vi "HFRR ADV v041.vi"() -> ()   [LabVIEW 2025] (continued)
                    n294 = call "ELAPSED TIMER VI - abort test.vi"("TARGET"=60.0, "RESET"=w401, "PAUSE"=FALSE) -> ("ELAPSED INDICATION"=w399:bool)  [unwired: 6 in, 2 out]
                    n295 = case shown="True" w399 {
                      frame False {
                      }
                      frame True {
                        n296 = stacked-sequence {
                          frame #0 {
                            w404 = FALSE
                            n297 = local write "RUN"(w404) -> ()
                            n298 = local write "Auto Start Test"(w404) -> ()
                          }
                          frame #1 {
                            n299 = One Button Dialog(message="Test stopped due to a communication error. Reconnect the C1 and C2 cables.") -> ()  [unwired: 1 in, 1 out]
                          }
                        }
                      }
                    }
                  }
                }
              }
            }
          }
          frame Enabled {
          }
        }
        n300 = Get Date/Time In Seconds() -> (seconds since 1Jan1904=w385:timestamp)
        n301 = Format Into String(format string="%<%I:%M:%S:%p %d:%B:%Y>T", w385) -> (resulting string=→"Time Stamp":string)  [unwired: 2 in, 1 out]
        n302 = local read "Service Password enable"() -> (w377:bool)
        n303 = local read "FILE"() -> (w382:string)
        n304 = call <vilib>:"Trim Whitespace.vi"("string"=w382) -> ("trimmed string"=w381:string)  [unwired: 1 in]
        n305 = String Length(string=w381) -> (length=w380:i32)
        n306 = Greater?(x=w380, y=1) -> (0:w378:bool)
        n307 = case shown="False" w378 {
          tunnel: w377 -> [w406 _]
          frame False {
            n308 = case shown="False" w406 {
              frame True {
                w407 = "Test Start In Service Mode" ("Tip Strip")
                w408 = T19."Enabled" ("Disabled")
                n309 = property on="Auto Start Test" class="Bool (strict)"("DisabledEnum"=w408, "TipStrip"=w407) -> ()  [unwired: 2 in, 2 out]
                n310 = property on="RUN" class="Bool (strict)"("DisabledEnum"=w408, "TipStrip"=w407) -> ()  [unwired: 2 in, 2 out]
              }
              frame False {
                w409 = "Enter File Name to Start Test" ("Tip Strip")
                w410 = T19."Disabled and Grayed Out" ("Disabled")
                n311 = property on="Auto Start Test" class="Bool (strict)"("DisabledEnum"=w410, "TipStrip"=w409) -> ()  [unwired: 2 in, 2 out]
                n312 = property on="RUN" class="Bool (strict)"("DisabledEnum"=w410, "TipStrip"=w409) -> ()  [unwired: 2 in, 2 out]
              }
            }
          }
          frame True {
            w411 = "" ("Tip Strip")
            w412 = T19."Enabled" ("Disabled")
            n313 = property on="Auto Start Test" class="Bool (strict)"("DisabledEnum"=w412, "TipStrip"=w411) -> ()  [unwired: 2 in, 2 out]
            n314 = property on="RUN" class="Bool (strict)"("DisabledEnum"=w412, "TipStrip"=w411) -> ()  [unwired: 2 in, 2 out]
          }
        }
      }
      event "RUN": Value Change {
        n315 = event-data() -> ()  [unwired: 1 in, 6 out]
        n316 = local read "RUN"() -> (w414:bool)
        n317 = case shown="False" w414 {
          frame False {
            n318 = flat-sequence {
              frame #0 {
                n319 = local write "START TEMP"(FALSE ("START TEMP")) -> ()
              }
              frame #1 {
                n320 = Wait (ms)(milliseconds to wait=u32 1500) -> ()  [unwired: 1 out]
              }
              frame #2 {
                n321 = local write "Humidity 2"(TRUE ("Humidity")) -> ()
              }
              frame #3 {
                n322 = local write "Due Write"("VC;0") -> ()
              }
              frame #4 {
                n323 = Wait (ms)(milliseconds to wait=u32 1500) -> ()  [unwired: 1 out]
              }
              frame #5 {
                w424 = T19."Enabled" ("Disabled")
                (unwired) T26."Imaging" ("Main Dashboard Buttons")
                (unwired) T21."Adv Scar" ("Main Tab")
                w426 = "" ("FILE")
                n324 = local write "measured_stroke"(0.0 ("measured_stroke")) -> ()
                n325 = local write "Due Write"("VC;0") -> ()
                n326 = local write "FILE"(w426) -> ()
                n327 = local write "Batch Ref Num :"(w426) -> ()
                n328 = local write "Fuel Discription :"(w426) -> ()
                n329 = local write "Main Tab"(T2."Adv Scar" ("Main Tab")) -> ()
                n330 = local write "Remarks :"(w426) -> ()
                n331 = local write "Main Dashboard Buttons"(T1."Imaging" ("Main Dashboard Buttons")) -> ()
                n332 = local write "TEST FILE NAM,E SAVED"(FALSE ("TEST FILE NAM,E SAVED")) -> ()
                n333 = property on="Stroke ( mm )" class="WFChart (strict)"("History Data"=cluster{"y":dbl, dbl, "y":dbl}[] []) -> ()  [unwired: 2 in, 2 out]
                n334 = property on="Auto Start Test" class="Bool (strict)"("Visible"=TRUE) -> ()  [unwired: 2 in, 2 out]
                n335 = property on="FRICVALZ 2" class="Bool (strict)"("DisabledEnum"=w424) -> ()  [unwired: 2 in, 2 out]
                n336 = property on="FRICVALZ 4" class="Bool (strict)"("DisabledEnum"=w424) -> ()  [unwired: 2 in, 2 out]
                n337 = property on="FRICVALZ 3" class="Bool (strict)"("DisabledEnum"=w424) -> ()  [unwired: 2 in, 2 out]
              }
            }
          }
          frame True {
            n338 = stacked-sequence {
              frame #0 {
                n339 = local write "Due Write"("DAC;200") -> ()
              }
              frame #1 {
                n340 = Wait (ms)(milliseconds to wait=u32 1500) -> ()  [unwired: 1 out]
              }
              frame #2 {
                n341 = local write "Due Write"("DAC;200") -> ()
              }
              frame #3 {
                n342 = Wait (ms)(milliseconds to wait=u32 1500) -> ()  [unwired: 1 out]
              }
              frame #4 {
                n343 = local write "Due Write"("VC;1") -> ()
              }
              frame #5 {
                n344 = Wait (ms)(milliseconds to wait=u32 2000) -> ()  [unwired: 1 out]
              }
              frame #6 {
                n345 = local write "Due Write"("VC;1") -> ()
              }
              frame #7 {
                n346 = Wait (ms)(milliseconds to wait=u32 2000) -> ()  [unwired: 1 out]
              }
              frame #8 {
                w438 = T19."Disabled" ("Disabled")
                n347 = property on="Auto Start Test" class="Bool (strict)"("Visible"=FALSE) -> ()  [unwired: 2 in, 2 out]
                n348 = local write "START TEMP"(TRUE ("START TEMP")) -> ()
                n349 = property on="FRICVALZ 2" class="Bool (strict)"("DisabledEnum"=w438) -> ()  [unwired: 2 in, 2 out]
                n350 = property on="FRICVALZ 4" class="Bool (strict)"("DisabledEnum"=w438) -> ()  [unwired: 2 in, 2 out]
                n351 = property on="FRICVALZ 3" class="Bool (strict)"("DisabledEnum"=w438) -> ()  [unwired: 2 in, 2 out]
              }
            }
          }
        }
      }
      event "run test Calibration": Value Change {
        n352 = event-data() -> ()  [unwired: 1 in, 6 out]
        n353 = local read "run test Calibration"() -> (w440:bool)
        n354 = case shown="True" w440 {
          frame False {
            n355 = flat-sequence {
              frame #0 {
                n356 = local write "START TEMP"(FALSE ("START TEMP")) -> ()
              }
              frame #1 {
                n357 = Wait (ms)(milliseconds to wait=u32 1500) -> ()  [unwired: 1 out]
              }
              frame #2 {
              }
              frame #3 {
                n358 = local write "Due Write"("VC;0") -> ()
              }
              frame #4 {
                n359 = Wait (ms)(milliseconds to wait=u32 1500) -> ()  [unwired: 1 out]
              }
              frame #5 {
                n360 = local write "Due Write"("VC;0") -> ()
                n361 = local write "Friction Force Calibration Result Tab"(enum32{"Calibration Results", "Page 2"}."Calibration Results" ("Friction Force Calibration Result Tab")) -> ()
                n362 = property on="Friction Force Calibration Result Tab" class="TabCtl (strict)"("Visible"=TRUE) -> ()  [unwired: 2 in, 2 out]
              }
            }
          }
          frame True {
            n363 = flat-sequence {
              frame #0 {
                n364 = local write "Due Write"("VC;1") -> ()
              }
              frame #1 {
                n365 = Wait (ms)(milliseconds to wait=u32 2000) -> ()  [unwired: 1 out]
              }
              frame #2 {
                n366 = local write "Due Write"("VC;1") -> ()
              }
              frame #3 {
                n367 = Wait (ms)(milliseconds to wait=u32 2000) -> ()  [unwired: 1 out]
              }
              frame #4 {
                n368 = local write "START TEMP"(TRUE ("START TEMP")) -> ()
                n369 = local write "Friction Force Calibration Result Tab"(enum32{"Calibration Results", "Page 2"}."Calibration Results" ("Friction Force Calibration Result Tab")) -> ()
                n370 = property on="Friction Force Calibration Result Tab" class="TabCtl (strict)"("Visible"=TRUE) -> ()  [unwired: 2 in, 2 out]
              }
            }
          }
        }
      }
      event "Auto": Value Change {
        n371 = event-data() -> ()  [unwired: 1 in, 6 out]
        n372 = stacked-sequence {
          frame #0 {
            n373 = local write "FILE"("") -> ()
          }
          frame #1 {
            n374 = Get Date/Time In Seconds() -> (seconds since 1Jan1904=w460:timestamp)
            n375 = Format Into String(format string="%<%I_%M_%S_%p_%d_%B_%Y>T", w460) -> (resulting string=w459:string)  [unwired: 2 in, 1 out]
            n376 = local write "FILE"(w459) -> ()
          }
        }
        n377 = local read "Auto"() -> (w457:bool)
        n378 = Not(x=w457) -> (.not. x?=w456:bool)
        n379 = local write "Auto"(w456) -> ()
      }
      event "Auto Start Temp": Value Change {
        n380 = event-data() -> ()  [unwired: 1 in, 6 out]
        n381 = local read "Auto Start Test"() -> (w463:bool)
        n382 = case shown="False" w463 {
          frame False {
            n383 = stacked-sequence {
              frame #0 {
                n384 = local write "START TEMP"(FALSE ("START TEMP")) -> ()
              }
              frame #1 {
                n385 = Wait (ms)(milliseconds to wait=u32 2000) -> ()  [unwired: 1 out]
              }
              frame #2 {
                n386 = local write "Due Write"("VC;0") -> ()
              }
              frame #3 {
                n387 = Wait (ms)(milliseconds to wait=u32 2000) -> ()  [unwired: 1 out]
              }
              frame #4 {
                w474 = T19."Enabled" ("Disabled")
                (unwired) T26."Imaging" ("Main Dashboard Buttons")
                w475 = "" ("FILE")
                n388 = local write "Main Tab"(T2."Adv Scar" ("Main Tab")) -> ()
                n389 = local write "measured_stroke"(0.0 ("measured_stroke")) -> ()
                n390 = local write "Main Dashboard Buttons"(T1."Imaging" ("Main Dashboard Buttons")) -> ()
                n391 = property on="RUN" class="Bool (strict)"("Visible"=TRUE) -> ()  [unwired: 2 in, 2 out]
                n392 = local write "Due Write"("VC;0") -> ()
                n393 = local write "Humidity 2"(TRUE ("Humidity")) -> ()
                n394 = local write "TEST FILE NAM,E SAVED"(FALSE ("TEST FILE NAM,E SAVED")) -> ()
                n395 = local write "Fuel Discription :"(w475) -> ()
                n396 = local write "Batch Ref Num :"(w475) -> ()
                n397 = local write "Remarks :"(w475) -> ()
                n398 = local write "FILE"(w475) -> ()
                n399 = property on="FRICVALZ 2" class="Bool (strict)"("DisabledEnum"=w474) -> ()  [unwired: 2 in, 2 out]
                n400 = property on="FRICVALZ 4" class="Bool (strict)"("DisabledEnum"=w474) -> ()  [unwired: 2 in, 2 out]
                n401 = property on="FRICVALZ 3" class="Bool (strict)"("DisabledEnum"=w474) -> ()  [unwired: 2 in, 2 out]
              }
            }
          }
          frame True {
            n402 = stacked-sequence {
              frame #0 {
                n403 = local write "Due Write"("DAC;200") -> ()
              }
              frame #1 {
                n404 = Wait (ms)(milliseconds to wait=u32 1500) -> ()  [unwired: 1 out]
              }
              frame #2 {
                n405 = local write "Due Write"("DAC;200") -> ()
              }
              frame #3 {
                n406 = Wait (ms)(milliseconds to wait=u32 1000) -> ()  [unwired: 1 out]
              }
              frame #4 {
                n407 = local write "Due Write"("VC;1") -> ()
              }
              frame #5 {
                n408 = Wait (ms)(milliseconds to wait=u32 2000) -> ()  [unwired: 1 out]
              }
              frame #6 {
                n409 = local write "Due Write"("VC;1") -> ()
              }
              frame #7 {
                n410 = Wait (ms)(milliseconds to wait=u32 2000) -> ()  [unwired: 1 out]
              }
              frame #8 {
                w486 = T19."Disabled" ("Disabled")
                n411 = property on="RUN" class="Bool (strict)"("Visible"=FALSE) -> ()  [unwired: 2 in, 2 out]
                n412 = property on="FRICVALZ 2" class="Bool (strict)"("DisabledEnum"=w486) -> ()  [unwired: 2 in, 2 out]
                n413 = property on="FRICVALZ 4" class="Bool (strict)"("DisabledEnum"=w486) -> ()  [unwired: 2 in, 2 out]
                n414 = property on="FRICVALZ 3" class="Bool (strict)"("DisabledEnum"=w486) -> ()  [unwired: 2 in, 2 out]
                "START TEMP" <- TRUE
              }
            }
          }
        }
      }
      event "FILE", "USERNAME", "USER ID": Mouse Enter {
        n415 = event-data() -> ()  [unwired: 1 in, 4 out]
        n416 = dll-call lib="kernel32.dll" fn="Wow64DisableWow64FsRedirection"("OldValue"=0) -> (error out=w493:errorcluster, "OldValue"=w491:i32)  [unwired: 4 in, 1 out]
        n417 = call <vilib>:"System Exec.vi"("run minimized? (F)"=TRUE, "error in (no error)"=w493, "command line"="C:\\Program Files\\Common Files\\Microsoft Shared\\Ink\\TabTip.exe") -> ("error out"=w492:errorcluster)  [unwired: 5 in, 3 out]
        n418 = dll-call lib="kernel32.dll" fn="Wow64EnableWow64FsRedirection"(error in=w492, "OldValue"=w491) -> ()  [unwired: 4 in, 2 out]
      }
      event "EDIT": Value Change {
        n419 = event-data() -> ()  [unwired: 1 in, 6 out]
        n420 = local read "EDIT"() -> (w494:bool)
        n421 = case shown="False" w494 {
          frame False {
            n422 = control-ref of="This VI"() -> (w511:refnum<vi>)
            n423 = property class="VI"(reference=w511) -> (reference out=w502:refnum<vi>, error out=w506:errorcluster, "Panel"=w510:refnum<vi>)  [unwired: 1 in]
            n424 = property class="Pnl"(reference=w510, error in=w506) -> (reference out=w504:refnum<vi>, error out=w507:errorcluster, "Panes[]"=w509:refnum<vi>[])
            n425 = for {
              tunnel: w509 -> [w517] mode=indexing
              tunnel: T24."Always Off" ("Horizontal Scrollbar Visibility") -> [w516]
              tunnel: w507 -> [w513]
              tunnel: [w512] -> w505
              n426 = property class="Pane"(reference=w517, error in=w513, "HorizScrollbarVisibility"=w516) -> (reference out=w514:refnum<vi>, error out=w515:errorcluster)
              n427 = Close Reference(reference=w514, error in (no error)=w515) -> (error out=w512:errorcluster)
            }
            n428 = Close Reference(reference=w504, error in (no error)=w505) -> (error out=w503:errorcluster)
            n429 = Close Reference(reference=w502, error in (no error)=w503) -> (error out=w497:errorcluster)
            "error out 7" <- w497
            n430 = call <vilib>:"Clear Errors.vi"("error in (no error)"=w497) -> ("error out"=w496:errorcluster)  [unwired: 5 in, 1 out]
            n431 = local write "Service Password enable"(FALSE ("Service Password enable")) -> ()
            n432 = call <userlib>:"Fit VI window to Largest Dec.vi"("error in (no error)"=w496, "border spacing (2 px)"=1) -> ("error out"=w501:errorcluster, "dup VI Ref"=w499:refnum<vi>)  [unwired: 4 in]
            n433 = invoke on="Invoke Node" class="VI" method="FP.Run-Time Position.Maximized"(reference=w499, error in=w501) -> (error out=w500:errorcluster)  [unwired: 2 in, 3 out]
            n434 = call <vilib>:"Clear Errors.vi"("error in (no error)"=w500) -> ()  [unwired: 5 in, 2 out]
          }
          frame True {
          }
        }
      }
      event "Heater Button": Value Change {
        n435 = event-data() -> ()  [unwired: 1 in, 6 out]
        n436 = local read "Heater Button"() -> (w518:bool)
        n437 = case shown="True" w518 {
          frame True {
            n438 = stacked-sequence {
              frame #0 {
                n439 = Wait (ms)(milliseconds to wait=u32 1500) -> ()  [unwired: 1 out]
              }
              frame #1 {
                n440 = local read "Set Temp"() -> (w520:dbl)
                n441 = Number To Fractional String(number=w520, precision (6)=i16 2) -> (F-format string=w523:string)  [unwired: 2 in]
                n442 = Concatenate Strings("ST;" ("Command"), w523) -> (w522:string)
                n443 = local write "Due Write"(w522) -> ()
              }
              frame #2 {
                n444 = Wait (ms)(milliseconds to wait=u32 1500) -> ()  [unwired: 1 out]
              }
              frame #3 {
                n445 = local write "Due Write"("HE;1" ("Command")) -> ()
              }
              frame #4 {
                n446 = Wait (ms)(milliseconds to wait=u32 1500) -> ()  [unwired: 1 out]
              }
              frame #5 {
                n447 = stacked-sequence {
                  frame #0 {
                    n448 = Wait (ms)(milliseconds to wait=u32 1500) -> ()  [unwired: 1 out]
                  }
                  frame #1 {
                    n449 = local read "Set Temp"() -> (w529:dbl)
                    n450 = Number To Fractional String(number=w529, precision (6)=i16 2) -> (F-format string=w532:string)  [unwired: 2 in]
                    n451 = Concatenate Strings("ST;" ("Command"), w532) -> (w531:string)
                    n452 = local write "Due Write"(w531) -> ()
                  }
                  frame #2 {
                    n453 = Wait (ms)(milliseconds to wait=u32 1500) -> ()  [unwired: 1 out]
                  }
                  frame #3 {
                    n454 = local write "Due Write"("HE;1" ("Command")) -> ()
                  }
                  frame #4 {
                    n455 = Wait (ms)(milliseconds to wait=u32 1500) -> ()  [unwired: 1 out]
                  }
                }
              }
            }
          }
          frame False {
            n456 = stacked-sequence {
              frame #0 {
                n457 = Wait (ms)(milliseconds to wait=u32 1500) -> ()  [unwired: 1 out]
              }
              frame #1 {
                n458 = Concatenate Strings("ST;" ("Command"), "0" ("string")) -> (w539:string)
                n459 = local write "Due Write"(w539) -> ()
              }
              frame #2 {
                n460 = Wait (ms)(milliseconds to wait=u32 1500) -> ()  [unwired: 1 out]
              }
              frame #3 {
                n461 = local write "Due Write"("HE;0" ("Command")) -> ()
              }
              frame #4 {
                n462 = Wait (ms)(milliseconds to wait=u32 1500) -> ()  [unwired: 1 out]
              }
            }
          }
        }
      }
      event "Headen Service Button": Value Change {
        n463 = event-data() -> ()  [unwired: 1 in, 6 out]
        n464 = local read "Headen Service Button"() -> (w544:bool)
        n465 = case shown="True" w544 {
          frame False {
            n466 = property on="Password 3" class="Clust (strict)"("Visible"=FALSE) -> ()  [unwired: 2 in, 2 out]
            n467 = property on="Service Password Log" class="Str"("Visible"=FALSE) -> ()  [unwired: 2 in, 2 out]
          }
          frame True {
            n468 = property on="Password 3" class="Clust (strict)"("Visible"=TRUE) -> ()  [unwired: 2 in, 2 out]
            n469 = property on="Service Password Log" class="Str"("Visible"=TRUE) -> ()  [unwired: 2 in, 2 out]
          }
        }
      }
      event "Password 3.Service Password": Value Change {
        n470 = event-data() -> ()  [unwired: 1 in, 6 out]
        n471 = Unbundle By Name("Password 3") -> ("Service Password"=w551:string)
        n472 = call <vilib>:"Trim Whitespace.vi"("string"=w551) -> ("trimmed string"=w549:string)  [unwired: 1 in]
        n473 = Equal?(x=w549, y="Service@123") -> (x = y?=w550:bool)
        n474 = case shown="False" w550 {
          selector: w550 -> [w554 w556]
          frame False {
            n475 = local write "Service Password enable"(w554) -> ()
            n476 = property on="Service Password Log" class="Str"("Visible"=TRUE) -> ()  [unwired: 2 in, 2 out]
          }
          frame True {
            n477 = property on="Service Password Log" class="Str"("Visible"=FALSE) -> ()  [unwired: 2 in, 2 out]
            "Service Password enable" <- w556
          }
        }
      }
      event "Sign In": Value Change {
        w558 = FALSE ("Visible")
        n478 = event-data() -> ()  [unwired: 1 in, 6 out]
        n479 = property on="About" class="Clust (strict)"("Visible"=w558) -> ()  [unwired: 2 in, 2 out]
        n480 = property on="Password 3" class="Clust (strict)"("Visible"=w558) -> ()  [unwired: 2 in, 2 out]
        n481 = property on="Service Password Log" class="Str"("Visible"=FALSE) -> ()  [unwired: 2 in, 2 out]
      }
      event "Info": Value Change {
        n482 = event-data() -> ()  [unwired: 1 in, 6 out]
        n483 = local read "Info"() -> (w560:bool)
        n484 = case shown="False" w560 {
          frame False {
            n485 = property on="About" class="Clust (strict)"("Visible"=FALSE) -> ()  [unwired: 2 in, 2 out]
          }
          frame True {
            n486 = property on="About" class="Clust (strict)"("Visible"=TRUE) -> ()  [unwired: 2 in, 2 out]
          }
        }
      }
      event "Calibration": Value Change {
        n487 = event-data() -> ()  [unwired: 1 in, 6 out]
        n488 = local read "Calibration"() -> (w564:bool)
        n489 = case shown="False" w564 {
          frame False {
            n490 = property on="Calibration 2" class="TabCtl (strict)"("Visible"=FALSE) -> ()  [unwired: 2 in, 2 out]
            n491 = local write "Cal Password"("" ("Cal Password")) -> ()
          }
          frame True {
            n492 = property on="Calibration 2" class="TabCtl (strict)"("Visible"=TRUE) -> ()  [unwired: 2 in, 2 out]
            n493 = local write "Cal Password"("" ("Cal Password")) -> ()
          }
        }
        n494 = property on="Wrong Password" class="Str"("Visible"=FALSE) -> ()  [unwired: 2 in, 2 out]
      }
      event "Cal Password": Value Change {
        n495 = event-data() -> ()  [unwired: 1 in, 6 out]
        n496 = local read "Cal Password"() -> (w572:string)
        n497 = call <vilib>:"Trim Whitespace.vi"("string"=w572) -> ("trimmed string"=w571:string)  [unwired: 1 in]
        n498 = Equal?(x=w571, y="Cal@321") -> (x = y?=w569:bool)
        n499 = case shown="True" w569 {
          frame False {
            n500 = property on="Wrong Password" class="Str"("Visible"=TRUE) -> ()  [unwired: 2 in, 2 out]
          }
          frame True {
            n501 = property on="Wrong Password" class="Str"("Visible"=FALSE) -> ()  [unwired: 2 in, 2 out]
            n502 = local write "Main Tab"(T2."About" ("Main Tab")) -> ()
            n503 = local write "Cal Password"("" ("Cal Password")) -> ()
            n504 = local write "Main Dashboard Buttons"(T1."About" ("Main Dashboard Buttons")) -> ()
            n505 = property on="Calibration 2" class="TabCtl (strict)"("Visible"=FALSE) -> ()  [unwired: 2 in, 2 out]
            n506 = local write "Calibration"(FALSE ("Calibration")) -> ()
          }
        }
      }
      event "Calibration Selection": Value Change {
        n507 = event-data() -> ()  [unwired: 1 in, 6 out]
        n508 = local read "Calibration Selection"() -> (w581:T8)
        n509 = case shown="\"Stroke Calibration\"" w581 {
          tunnel: [T7."Stroke" ("Main Calibration Tab") T7."Friction" ("Main Calibration Tab") T7."Main" ("Main Calibration Tab") T7."Temperature" ("Main Calibration Tab")] -> w580
          frame "Stroke Calibration" {
          }
          frame "Friction Force Calibration" {
          }
          frame Default {
          }
          frame "Temperature Calibration" {
          }
        }
        n510 = local write "Main Calibration Tab"(w580) -> ()
      }
      event "Back Stroke": Value Change {
        n511 = event-data() -> ()  [unwired: 1 in, 6 out]
        n512 = local write "Main Stroke Tab"(T9."Step 1" ("Main Stroke Tab")) -> ()
        n513 = local write "Main Calibration Tab"(T7."Main" ("Main Calibration Tab")) -> ()
        n514 = local write "Back Stroke"(FALSE ("Back Stroke")) -> ()
        n515 = local write "Calibration Selection"(T8."Default" ("Calibration Selection")) -> ()
      }
      event "Step 2 Back": Value Change {
        n516 = event-data() -> ()  [unwired: 1 in, 6 out]
        n517 = local write "Main Stroke Tab"(T9."Step 1" ("Main Stroke Tab")) -> ()
        n518 = local write "Step 2 Back"(FALSE ("Back Stroke")) -> ()
        n519 = local write "Calibration Selection"(T8."Default" ("Calibration Selection")) -> ()
      }
      event "Step 3 Back": Value Change {
        n520 = event-data() -> ()  [unwired: 1 in, 6 out]
        n521 = local write "Main Stroke Tab"(T9."Step 2" ("Main Stroke Tab")) -> ()
        n522 = local write "Step 3 Back"(FALSE ("Back Stroke")) -> ()
        n523 = local write "Calibration Selection"(T8."Default" ("Calibration Selection")) -> ()
      }
      event "Step 4 Back": Value Change {
        n524 = event-data() -> ()  [unwired: 1 in, 6 out]
        n525 = local write "Main Stroke Tab"(T9."Step 3" ("Main Stroke Tab")) -> ()
        n526 = local write "Step 4 Back"(FALSE ("Back Stroke")) -> ()
        n527 = local write "Calibration Selection"(T8."Default" ("Calibration Selection")) -> ()
      }
      event "Step 5 Back": Value Change {
        n528 = event-data() -> ()  [unwired: 1 in, 6 out]
        n529 = local write "Main Stroke Tab"(T9."Step 4" ("Main Stroke Tab")) -> ()
        n530 = local write "Step 5 Back"(FALSE ("Back Stroke")) -> ()
        n531 = local write "Calibration Selection"(T8."Default" ("Calibration Selection")) -> ()
      }
      event "Step 6 Back": Value Change {
        n532 = event-data() -> ()  [unwired: 1 in, 6 out]
        n533 = local write "Main Stroke Tab"(T9."Step 5" ("Main Stroke Tab")) -> ()
        n534 = local write "Step 6 Back"(FALSE ("Back Stroke")) -> ()
        n535 = local write "Calibration Selection"(T8."Default" ("Calibration Selection")) -> ()
      }
      event "Back Stroke step 7": Value Change {
        n536 = event-data() -> ()  [unwired: 1 in, 6 out]
        n537 = local write "Main Stroke Tab"(T9."Step 5" ("Main Stroke Tab")) -> ()
        n538 = local write "Back Stroke step 7"(FALSE ("Back Stroke")) -> ()
        n539 = local write "Calibration Selection"(T8."Default" ("Calibration Selection")) -> ()
      }
      event "Back Stroke step 8": Value Change {
        n540 = event-data() -> ()  [unwired: 1 in, 6 out]
        n541 = local write "Main Stroke Tab"(T9."Step 7" ("Main Stroke Tab")) -> ()
        n542 = local write "Back Stroke step 8"(FALSE ("Back Stroke")) -> ()
        n543 = local write "Calibration Selection"(T8."Default" ("Calibration Selection")) -> ()
      }
      event "Back Stroke 8": Value Change {
        n544 = event-data() -> ()  [unwired: 1 in, 6 out]
        n545 = local write "MOVE CARRIAGE TO"(1.0 ("MOVE CARRIAGE TO")) -> ()
        n546 = local write "Main Stroke Tab"(T9."Step 1" ("Main Stroke Tab")) -> ()
        n547 = local write "Calibration Selection"(T8."Default" ("Calibration Selection")) -> ()
        n548 = local write "Back Stroke 8"(FALSE ("Back Stroke 8")) -> ()
      }
      event "Continue Stroke": Value Change {
        n549 = event-data() -> ()  [unwired: 1 in, 6 out]
        n550 = local write "Main Stroke Tab"(T9."Step 2" ("Main Stroke Tab")) -> ()
        n551 = local write "Continue Stroke"(FALSE ("Continue Stroke")) -> ()
      }
      event "Continue Stroke step 2": Value Change {
        n552 = event-data() -> ()  [unwired: 1 in, 6 out]
        n553 = local write "Main Stroke Tab"(T9."Step 3" ("Main Stroke Tab")) -> ()
        n554 = local write "Continue Stroke step 2"(FALSE ("Continue Stroke")) -> ()
      }
      event "Continue Stroke step 3": Value Change {
        n555 = event-data() -> ()  [unwired: 1 in, 6 out]
        n556 = local write "Main Stroke Tab"(T9."Step 4" ("Main Stroke Tab")) -> ()
        n557 = local write "Continue Stroke step 3"(FALSE ("Continue Stroke")) -> ()
      }
      event "Continue Stroke step 4": Value Change {
        n558 = event-data() -> ()  [unwired: 1 in, 6 out]
        n559 = local write "Main Stroke Tab"(T9."Step 5" ("Main Stroke Tab")) -> ()
        n560 = local write "Continue Stroke step 4"(FALSE ("Continue Stroke")) -> ()
      }
      event "Continue Stroke step 5": Value Change {
        n561 = event-data() -> ()  [unwired: 1 in, 6 out]
        n562 = local write "Main Stroke Tab"(T9."Step 7" ("Main Stroke Tab")) -> ()
        n563 = local write "Continue Stroke step 5"(FALSE ("Continue Stroke")) -> ()
      }
      event "Continue Stroke step 6": Value Change {
        n564 = event-data() -> ()  [unwired: 1 in, 6 out]
        n565 = local write "Main Stroke Tab"(T9."Step 7" ("Main Stroke Tab")) -> ()
        n566 = local write "Continue Stroke step 6"(FALSE ("Continue Stroke")) -> ()
      }
      event "Continue Stroke step 7": Value Change {
        w629 = FALSE ("0.2mm")
        n567 = event-data() -> ()  [unwired: 1 in, 6 out]
        n568 = local write "0.4 mm"(w629) -> ()
        n569 = local write "0.6 mm"(w629) -> ()
        n570 = local write "1.0 mm"(w629) -> ()
        n571 = local write "1.2 mm"(w629) -> ()
        n572 = local write "0.2 2"(w629) -> ()
        n573 = local write "0.4 2"(w629) -> ()
        n574 = local write "0.6 2"(w629) -> ()
        n575 = local write "0.8 2"(w629) -> ()
        n576 = local write "1.0 2"(w629) -> ()
        n577 = local write "1.2"(w629) -> ()
        n578 = local write "0.2mm"(w629) -> ()
        n579 = local write "0.8mm"(w629) -> ()
        n580 = local write "Main Stroke Tab"(T9."Step 8" ("Main Stroke Tab")) -> ()
        n581 = local write "Continue Stroke step 7"(FALSE ("Continue Stroke")) -> ()
        n582 = local write "Stroke Test Complete"(T10."Test Progress" ("Stroke Test Complete")) -> ()
        "Position Measurment Temp" <- 4.0 ("Position Measurment Temp")
        "Calibration Tare" <- TRUE ("Calibration Tare")
        "MOVE CARRIAGE TO" <- 1.0 ("MOVE CARRIAGE TO")
      }
      event "Continue Stroke step 8": Value Change {
        n583 = event-data() -> ()  [unwired: 1 in, 6 out]
        n584 = local read "LVDT STROKE  Calibration"() -> (w634:dbl)
        n585 = local read "Position Measurment Temp"() -> (w635:dbl)
        n586 = case shown="7" w635 {
          selector: w635 -> [w640 w645 w650 w655 _ w663 w666 w667]
          tunnel: w634 -> [w636 w641 w646 w651 w657 w660 _ _]
          frame 0, Default {
            w638 = TRUE ("0.2mm")
            n587 = Increment(x=w640) -> (x+1=w639:i32)
            n588 = local write "Position Measurment Temp"(w639) -> ()
            n589 = local write "0.2mm"(w638) -> ()
            n590 = local write "0.2 2"(w638) -> ()
            n591 = local write "MOVE CARRIAGE TO"(1.0 ("MOVE CARRIAGE TO")) -> ()
            "Calibration 0.2" <- w636
          }
          frame 1 {
            w643 = TRUE ("0.4 mm")
            n592 = Increment(x=w645) -> (x+1=w644:i32)
            n593 = local write "Calibration 0.4"(w641) -> ()
            n594 = local write "Position Measurment Temp"(w644) -> ()
            n595 = local write "0.4 mm"(w643) -> ()
            n596 = local write "MOVE CARRIAGE TO"(0.6 ("MOVE CARRIAGE TO")) -> ()
            n597 = local write "0.4 2"(w643) -> ()
          }
          frame 2 {
            w648 = TRUE ("0.6 mm")
            n598 = Increment(x=w650) -> (x+1=w649:i32)
            n599 = local write "Calibration 0.6"(w646) -> ()
            n600 = local write "Position Measurment Temp"(w649) -> ()
            n601 = local write "0.6 2"(w648) -> ()
            n602 = local write "0.6 mm"(w648) -> ()
            n603 = local write "MOVE CARRIAGE TO"(0.8 ("MOVE CARRIAGE TO")) -> ()
          }
          frame 3 {
            w652 = TRUE ("0.6 mm")
            n604 = Increment(x=w655) -> (x+1=w654:i32)
            n605 = local write "Position Measurment Temp"(w654) -> ()
            n606 = local write "MOVE CARRIAGE TO"(1.0 ("MOVE CARRIAGE TO")) -> ()
            n607 = local write "0.8mm"(w652) -> ()
            n608 = local write "0.8 2"(w652) -> ()
            "Calibration 0.8" <- w651
          }
          frame 4 {
            w658 = TRUE ("0.6 mm")
            n609 = local write "Position Measurment Temp"(6.0 ("Position Measurment Temp")) -> ()
            n610 = local write "MOVE CARRIAGE TO"(1.0 ("MOVE CARRIAGE TO")) -> ()
            n611 = local write "1.0 mm"(w658) -> ()
            n612 = local write "1.0 2"(w658) -> ()
            "Calibration 1.0" <- w657
          }
          frame 5 {
            w661 = TRUE ("0.6 mm")
            n613 = Increment(x=w663) -> (x+1=w662:i32)
            n614 = local write "Position Measurment Temp"(w662) -> ()
            n615 = local write "1.2 mm"(w661) -> ()
            n616 = local write "1.2"(w661) -> ()
            "Calibration 1.2" <- w660
          }
          frame 6 {
            n617 = Increment(x=w666) -> (x+1=w665:i32)
            n618 = local write "Position Measurment Temp"(w665) -> ()
            n619 = local write "Stroke Test Complete"(T10."Stroke Points Completed" ("Stroke Test Complete")) -> ()
          }
          frame 7 {
            n620 = stacked-sequence {
              tunnel: w667 -> [w668 _ _]
              frame #0 {
                n621 = Increment(x=w668) -> (x+1=w669:i32)
                n622 = local write "Main Stroke Tab"(T9."Step 9" ("Main Stroke Tab")) -> ()
                n623 = local write "Position Measurment Temp"(w669) -> ()
                n624 = Insert Into Array(array=dbl[] [], new element #1=0.2 ("new element/subarray"), new element #2=0.4 ("new element/subarray"), new element #3=0.6 ("new element/subarray"), new element #4=0.8 ("new element/subarray"), new element #5=1.0 ("new element/subarray"), new element #6=1.2 ("new element/subarray")) -> (→"1D stroke":dbl[])  [unwired: 1 in]
                n625 = local read "Calibration 0.2"() -> (w676:dbl)
                n626 = local read "Calibration 0.4"() -> (w675:dbl)
                n627 = local read "Calibration 0.6"() -> (w674:dbl)
                n628 = local read "Calibration 0.8"() -> (w673:dbl)
                n629 = local read "Calibration 1.0"() -> (w672:dbl)
                n630 = local read "Calibration 1.2"() -> (w671:dbl)
                n631 = Insert Into Array(array=dbl[] [], new element #1=w676, new element #2=w675, new element #3=w674, new element #4=w673, new element #5=w672, new element #6=w671) -> (→"Calibrated Voltage Value":dbl[])  [unwired: 1 in]
              }
              frame #1 {
                n632 = local read "calibration values"() -> (w699:dbl[])
                n633 = local read "Calibrated Voltage Value"() -> (w701:dbl[])
                n634 = Index Array(array=w699, index #1=1 ("index"), index #2=3 ("index"), index #3=5 ("index"), index #4=7 ("index"), index #5=9 ("index"), index #6=11 ("index")) -> (element #1=w692:dbl, element #2=w691:dbl, element #3=w690:dbl, element #4=w689:dbl, element #5=w688:dbl, element #6=w687:dbl)
                n635 = local read "1D stroke"() -> (w702:dbl[])
                n636 = for {
                  tunnel: [w711] -> w700 mode=indexing
                  tunnel: w702 -> [w710] mode=indexing
                  tunnel: w701 -> [w709] mode=indexing
                  tunnel: w692 -> [w708]
                  tunnel: w691 -> [w707]
                  tunnel: w690 -> [w706]
                  tunnel: w689 -> [w705]
                  tunnel: w688 -> [w704]
                  tunnel: w687 -> [w703]
                  n637 = formula code="if (stroke == 0.2)\n{\n    if ((voltage >= REF_02 - 0.2) && (voltage <= REF_02 + 0.2))\n        status = 1;\n    else\n        status = 0;\n}\nelse if (stroke == 0.4)\n{\n    if ((voltage >= REF_04 - 0.2) && (voltage <= REF_04 + 0.2))\n        status = 1;\n    else\n        status = 0;\n}\nelse if (stroke == 0.6)\n{\n    if ((voltage >= REF_06 - 0.2) && (voltage <= REF_06 + 0.2))\n        status = 1;\n    else\n        status = 0;\n}\nelse if (stroke == 0.8)\n{\n    if ((voltage >= REF_08 - 0.2) && (voltage <= REF_08 + 0.2))\n        status = 1;\n    else\n        status = 0;\n}\nelse if (stroke == 1.0)\n{\n    if ((voltage >= REF_10 - 0.4) && (voltage <= REF_10 + 0.4))\n        status = 1;\n    else\n        status = 0;\n}\nelse if (stroke == 1.2)\n{\n    if ((voltage >= REF_12 - 0.2) && (voltage <= REF_12 + 0.2))\n        status = 1;\n    else\n        status = 0;\n}\nelse\n{\n    status = 0;\n}"("stroke"=w710, "voltage"=w709, "REF_02"=w708, "REF_04"=w707, "REF_06"=w706, "REF_08"=w705, "REF_10"=w704, "REF_12"=w703) -> ("status"=w711:dbl)
                }
                "Status" <- w700
              }
              frame #2 {
                w718 = 1.0
                n638 = local read "Status"() -> (w725:dbl[])
                n639 = Index Array(array=w725) -> (element #1=w724:dbl, element #2=w723:dbl, element #3=w722:dbl, element #4=w721:dbl, element #5=w720:dbl, element #6=w719:dbl)  [unwired: 6 in]
                n640 = Equal?(x=w723, y=w718) -> (x = y?=w716:bool)
                n641 = Equal?(x=w722, y=w718) -> (x = y?=w715:bool)
                n642 = Equal?(x=w721, y=w718) -> (x = y?=w714:bool)
                n643 = Equal?(x=w720, y=w718) -> (x = y?=w713:bool)
                n644 = Equal?(x=w719, y=w718) -> (x = y?=w712:bool)
                n645 = Equal?(x=w724, y=w718) -> (x = y?=w717:bool)
                n646 = case shown="True" w717 {
                  selector: w717 -> [w736 w737]
                  frame True {
                    n647 = local write "Point 1 - 0.2 mm"(w736) -> ()
                    n648 = property on="Point 1 - 0.2 mm" class="Bool"("Caption.Visible"=w736) -> ()  [unwired: 2 in, 2 out]
                  }
                  frame False {
                    n649 = local write "Point 1 - 0.2 mm"(w737) -> ()
                    n650 = property on="Point 1 - 0.2 mm" class="Bool"("Caption.Visible"=w737) -> ()  [unwired: 2 in, 2 out]
                  }
                }
                n651 = case shown="True" w716 {
                  selector: w716 -> [w734 w735]
                  frame True {
                    n652 = local write "Point 2 - 0.4 mm"(w734) -> ()
                    n653 = property on="Point 2 - 0.4 mm" class="Bool"("Caption.Visible"=w734) -> ()  [unwired: 2 in, 2 out]
                  }
                  frame False {
                    n654 = local write "Point 2 - 0.4 mm"(w735) -> ()
                    n655 = property on="Point 2 - 0.4 mm" class="Bool"("Caption.Visible"=w735) -> ()  [unwired: 2 in, 2 out]
                  }
                }
                n656 = case shown="True" w713 {
                  selector: w713 -> [w728 w729]
                  frame True {
                    n657 = local write "Point 5 - 1.0 mm"(w728) -> ()
                    n658 = property on="Point 5 - 1.0 mm" class="Bool"("Caption.Visible"=w728) -> ()  [unwired: 2 in, 2 out]
                  }
                  frame False {
                    n659 = local write "Point 5 - 1.0 mm"(w729) -> ()
                    n660 = property on="Point 5 - 1.0 mm" class="Bool"("Caption.Visible"=w729) -> ()  [unwired: 2 in, 2 out]
                  }
                }
                n661 = case shown="True" w715 {
                  selector: w715 -> [w732 w733]
                  frame True {
                    n662 = local write "Point 3 - 0.6 mm"(w732) -> ()
                    n663 = property on="Point 3 - 0.6 mm" class="Bool"("Caption.Visible"=w732) -> ()  [unwired: 2 in, 2 out]
                  }
                  frame False {
                    n664 = local write "Point 3 - 0.6 mm"(w733) -> ()
                    n665 = property on="Point 3 - 0.6 mm" class="Bool"("Caption.Visible"=w733) -> ()  [unwired: 2 in, 2 out]
                  }
                }
                n666 = case shown="True" w714 {
                  selector: w714 -> [w730 w731]
                  frame True {
                    n667 = local write "Point 4 - 0.8 mm"(w730) -> ()
                    n668 = property on="Point 4 - 0.8 mm" class="Bool"("Caption.Visible"=w730) -> ()  [unwired: 2 in, 2 out]
                  }
                  frame False {
                    n669 = local write "Point 4 - 0.8 mm"(w731) -> ()
                    n670 = property on="Point 4 - 0.8 mm" class="Bool"("Caption.Visible"=w731) -> ()  [unwired: 2 in, 2 out]
                  }
                }
                n671 = case shown="True" w712 {
                  selector: w712 -> [w726 w727]
                  frame True {
                    n672 = local write "Point 6 - 1.2 mm"(w726) -> ()
                    n673 = property on="Point 6 - 1.2 mm" class="Bool"("Caption.Visible"=w726) -> ()  [unwired: 2 in, 2 out]
                  }
                  frame False {
                    n674 = local write "Point 6 - 1.2 mm"(w727) -> ()
                    n675 = property on="Point 6 - 1.2 mm" class="Bool"("Caption.Visible"=w727) -> ()  [unwired: 2 in, 2 out]
                  }
                }
              }
            }
          }
        }
      }
      event "Accept & Save": Value Change {
        n676 = event-data() -> ()  [unwired: 1 in, 6 out]
        n677 = flat-sequence {
          frame #0 {
            n678 = Get Date/Time In Seconds() -> (seconds since 1Jan1904=w740:timestamp)
            n679 = Format Into String(format string="%<%I:%M:%S:%p %d:%B:%Y>T", w740) -> (resulting string=w738:string)  [unwired: 2 in, 1 out]
            n680 = local write "STROKE CALIBRATION"(w738) -> ()
          }
          frame #1 {
            n681 = local write "Save Button"(TRUE ("Save Button")) -> ()
          }
          frame #2 {
            n682 = local write "MOVE CARRIAGE TO"(1.0 ("MOVE CARRIAGE TO")) -> ()
            n683 = local write "Main Calibration Tab"(T7."Main" ("Main Calibration Tab")) -> ()
            n684 = local write "Main Stroke Tab"(T9."Step 1" ("Main Stroke Tab")) -> ()
            n685 = local write "Calibration Selection"(T8."Default" ("Calibration Selection")) -> ()
            n686 = local write "Back Stroke 8"(FALSE ("Back Stroke 8")) -> ()
          }
        }
      }
      event "TEMPERATURE STEP Back 1", "TEMPERATURE STEP Back air Temp": Value Change {
        n687 = event-data() -> ()  [unwired: 1 in, 6 out]
        n688 = stacked-sequence {
          frame #0 {
            n689 = local write "Main Calibration Tab"(T7."Main" ("Main Calibration Tab")) -> ()
            n690 = local write "Temperature Selection"(T13."Default" ("Temperature Selection")) -> ()
          }
          frame #1 {
            n691 = Wait (ms)(milliseconds to wait=u32 1000) -> ()  [unwired: 1 out]
            n692 = local write "Calibration Selection"(T8."Default" ("Calibration Selection")) -> ()
          }
          frame #2 {
            n693 = local write "Due Write"("CAL;END" ("Command")) -> ()
          }
          frame #3 {
            n694 = Wait (ms)(milliseconds to wait=u32 2000) -> ()  [unwired: 1 out]
          }
          frame #4 {
            n695 = local write "Due Write"("CAL;END" ("Command")) -> ()
          }
        }
      }
      event "Temperature Continue Step 1": Value Change {
        n696 = event-data() -> ()  [unwired: 1 in, 6 out]
        n697 = stacked-sequence {
          frame #0 {
            n698 = Wait (ms)(milliseconds to wait=u32 1500) -> ()  [unwired: 1 out]
          }
          frame #1 {
            n699 = local write "Due Write"("CAL;START" ("Command")) -> ()
          }
          frame #2 {
            n700 = Wait (ms)(milliseconds to wait=u32 1500) -> ()  [unwired: 1 out]
          }
          frame #3 {
            n701 = local write "Due Write"("CAL;START" ("Command")) -> ()
          }
          frame #4 {
            n702 = Wait (ms)(milliseconds to wait=u32 2000) -> ()  [unwired: 1 out]
          }
          frame #5 {
          }
          frame #6 {
            n703 = Wait (ms)(milliseconds to wait=u32 2000) -> ()  [unwired: 1 out]
          }
          frame #7 {
            # "CAL;A1;<true_T>"
            n704 = local write "Due Write"("CAL;A1;0" ("Command")) -> ()
          }
          frame #8 {
            n705 = local write "Tab Control 4"(T12."Step 2" ("Tab Control 4")) -> ()
          }
        }
      }
      event "Temperature Continue Step air Step 1": Value Change {
        n706 = event-data() -> ()  [unwired: 1 in, 6 out]
        n707 = stacked-sequence {
          frame #0 {
            n708 = Wait (ms)(milliseconds to wait=u32 1500) -> ()  [unwired: 1 out]
          }
          frame #1 {
            n709 = local write "Due Write"("CAL;START" ("Command")) -> ()
          }
          frame #2 {
            n710 = Wait (ms)(milliseconds to wait=u32 1500) -> ()  [unwired: 1 out]
          }
          frame #3 {
            n711 = local write "Due Write"("CAL;START" ("Command")) -> ()
          }
          frame #4 {
            n712 = Wait (ms)(milliseconds to wait=u32 2000) -> ()  [unwired: 1 out]
          }
          frame #5 {
          }
          frame #6 {
            n713 = Wait (ms)(milliseconds to wait=u32 2000) -> ()  [unwired: 1 out]
          }
          frame #7 {
            # "CAL;A1;<true_T>"
            n714 = local write "Due Write"("CAL;A1;0" ("Command")) -> ()
          }
          frame #8 {
            n715 = local write "Tab Control 4"(T12."Air Step 2" ("Tab Control 4")) -> ()
          }
        }
      }
      event "Temperature Selection": Value Change {
        n716 = event-data() -> ()  [unwired: 1 in, 6 out]
        n717 = local read "Temperature Selection"() -> (w770:T13)
        n718 = case shown="\"Sample Temperature\"" w770 {
          frame "Air Temperature" {
            n719 = local write "Tab Control 4"(T12."Air Step 1" ("Tab Control 4")) -> ()
          }
          frame "Sample Temperature" {
            n720 = local write "Tab Control 4"(T12."Step 1" ("Tab Control 4")) -> ()
          }
          frame "Default", Default {
          }
        }
      }
      event "Temperature Continue Step 2": Value Change {
        n721 = event-data() -> ()  [unwired: 1 in, 6 out]
        n722 = stacked-sequence {
          frame #0 {
            n723 = stacked-sequence {
              frame #0 {
                n724 = Wait (ms)(milliseconds to wait=u32 1500) -> ()  [unwired: 1 out]
              }
              frame #1 {
                # "CAL;A1;<true_T>"
                n725 = local read "Sensor value"() -> (→"Sample 0deg temp":dbl)
                n726 = local write "Due Write"("CAL;A1;0" ("Command")) -> ()
              }
              frame #2 {
                n727 = Wait (ms)(milliseconds to wait=u32 1500) -> ()  [unwired: 1 out]
              }
              frame #3 {
                # "CAL;A1;<true_T>"
                n728 = local write "Due Write"("CAL;A1;0" ("Command")) -> ()
              }
              frame #4 {
              }
            }
          }
          frame #1 {
            n729 = local write "Tab Control 4"(T12."Step 3" ("Tab Control 4")) -> ()
          }
        }
      }
      event "Temperature Continue Air Step 2": Value Change {
        n730 = event-data() -> ()  [unwired: 1 in, 6 out]
        n731 = stacked-sequence {
          frame #0 {
            n732 = stacked-sequence {
              frame #0 {
                n733 = Wait (ms)(milliseconds to wait=u32 1000) -> ()  [unwired: 1 out]
              }
              frame #1 {
                # "CAL;A1;<true_T>"
                n734 = local write "Due Write"("CAL;A1;0" ("Command")) -> ()
              }
              frame #2 {
                n735 = Wait (ms)(milliseconds to wait=u32 1000) -> ()  [unwired: 1 out]
              }
              frame #3 {
                # "CAL;A1;<true_T>"
                n736 = local write "Due Write"("CAL;A1;0" ("Command")) -> ()
              }
              frame #4 {
                n737 = local read "Sensor value"() -> (→"Air 0deg temp":dbl)
              }
            }
          }
          frame #1 {
            n738 = local write "Tab Control 4"(T12."Air Step 3" ("Tab Control 4")) -> ()
          }
        }
      }
      event "Temperature Continue Step 3": Value Change {
        n739 = event-data() -> ()  [unwired: 1 in, 6 out]
        n740 = stacked-sequence {
          frame #0 {
            n741 = stacked-sequence {
              frame #0 {
                n742 = Wait (ms)(milliseconds to wait=u32 1500) -> ()  [unwired: 1 out]
              }
              frame #1 {
              }
              frame #2 {
              }
              frame #3 {
                # "CAL;A1;<true_T>"
                n743 = local write "Due Write"("CAL;A1;60" ("Command")) -> ()
              }
              frame #4 {
                n744 = Wait (ms)(milliseconds to wait=u32 1000) -> ()  [unwired: 1 out]
              }
              frame #5 {
                # "CAL;A1;<true_T>"
                n745 = local read "Sensor value"() -> (→"Sample 60deg temp":dbl)
                n746 = local write "Due Write"("CAL;A1;60" ("Command")) -> ()
              }
            }
          }
          frame #1 {
            n747 = local read "Sample 0deg temp"() -> (w799:dbl)
            n748 = local read "Sample 60deg temp"() -> (w798:dbl)
            n749 = Add(x=w798, y="Temperature diff") -> (x+y=w796:dbl)
            n750 = Subtract(x=w798, y="Temperature diff") -> (x-y=w795:dbl)
            n751 = Add(x=w799, y="Temperature diff") -> (x+y=w794:dbl)
            n752 = Subtract(x=w799, y="Temperature diff") -> (x-y=w793:dbl)
            n753 = In Range and Coerce(upper limit=w796, x=w798, lower limit=w795) -> (In Range?=w792:bool)  [unwired: 1 out]
            n754 = In Range and Coerce(upper limit=w794, x=w799, lower limit=w793) -> (In Range?=w791:bool)  [unwired: 1 out]
            n755 = And(x=w792, y=w791) -> (x .and. y?=w790:bool)
            n756 = case shown="True" w790 {
              frame False {
                n757 = property on="Accept & Save sample Temperature step 4" class="Bool (strict)"("DisabledEnum"=T19."Disabled" ("Disabled")) -> ()  [unwired: 2 in, 2 out]
                n758 = local write "Sample Temperature Calibration  2"(enum32{"True", "Fail"}."Fail" ("Sample Temperature Calibration  2")) -> ()
              }
              frame True {
                n759 = property on="Accept & Save sample Temperature step 4" class="Bool (strict)"("DisabledEnum"=T19."Enabled" ("Disabled")) -> ()  [unwired: 2 in, 2 out]
                n760 = local write "Sample Temperature Calibration  2"(enum32{"True", "Fail"}."True" ("Sample Temperature Calibration  2")) -> ()
              }
            }
          }
          frame #2 {
          }
          frame #3 {
          }
          frame #4 {
          }
          frame #5 {
          }
          frame #6 {
            # "CAL;END"
          }
          frame #7 {
          }
          frame #8 {
            # "CAL;END"
          }
          frame #9 {
            n761 = local write "Tab Control 4"(T12."Step 4" ("Tab Control 4")) -> ()
          }
        }
      }
      event "Accept & Save sample Temperature step 4": Value Change {
        n762 = event-data() -> ()  [unwired: 1 in, 6 out]
        n763 = stacked-sequence {
          frame #0 {
            n764 = local write "Due Write"("CAL;SAVE" ("Command")) -> ()
          }
          frame #1 {
            n765 = Wait (ms)(milliseconds to wait=u32 1000) -> ()  [unwired: 1 out]
          }
          frame #2 {
            n766 = local write "Due Write"("CAL;SAVE" ("Command")) -> ()
          }
          frame #3 {
            n767 = Wait (ms)(milliseconds to wait=u32 1000) -> ()  [unwired: 1 out]
          }
          frame #4 {
            n768 = local write "Due Write"("CAL;END" ("Command")) -> ()
          }
          frame #5 {
            n769 = Wait (ms)(milliseconds to wait=u32 1000) -> ()  [unwired: 1 out]
          }
          frame #6 {
            n770 = local write "Due Write"("CAL;END" ("Command")) -> ()
            n771 = local write "Temperature Selection"(T13."Default" ("Temperature Selection")) -> ()
            n772 = local write "Calibration Selection"(T8."Default" ("Calibration Selection")) -> ()
            n773 = local write "Tab Control 4"(T12."Main" ("Tab Control 4")) -> ()
            n774 = local write "Main Calibration Tab"(T7."Temperature" ("Main Calibration Tab")) -> ()
          }
          frame #7 {
            n775 = Get Date/Time In Seconds() -> (seconds since 1Jan1904=w818:timestamp)
            n776 = Format Into String(format string="%<%I:%M:%S:%p %d:%B:%Y>T", w818) -> (resulting string=w816:string)  [unwired: 2 in, 1 out]
            n777 = local write "TEMPERATURE CALIBRATION"(w816) -> ()
          }
          frame #8 {
            n778 = local write "Save Button"(TRUE ("Save Button")) -> ()
          }
        }
      }
      event "Accept & Save Air Temperature step 4": Value Change {
        n779 = event-data() -> ()  [unwired: 1 in, 6 out]
        n780 = stacked-sequence {
          frame #0 {
            n781 = local write "Due Write"("CAL;SAVE" ("Command")) -> ()
          }
          frame #1 {
            n782 = Wait (ms)(milliseconds to wait=u32 1000) -> ()  [unwired: 1 out]
          }
          frame #2 {
            n783 = local write "Due Write"("CAL;SAVE" ("Command")) -> ()
          }
          frame #3 {
            n784 = Wait (ms)(milliseconds to wait=u32 1000) -> ()  [unwired: 1 out]
          }
          frame #4 {
            n785 = local write "Due Write"("CAL;END" ("Command")) -> ()
          }
          frame #5 {
            n786 = Wait (ms)(milliseconds to wait=u32 1000) -> ()  [unwired: 1 out]
          }
          frame #6 {
            n787 = local write "Due Write"("CAL;END" ("Command")) -> ()
            n788 = local write "Tab Control 4"(T12."Main" ("Tab Control 4")) -> ()
            n789 = local write "Main Calibration Tab"(T7."Temperature" ("Main Calibration Tab")) -> ()
            n790 = local write "Temperature Selection"(T13."Default" ("Temperature Selection")) -> ()
            n791 = local write "Calibration Selection"(T8."Default" ("Calibration Selection")) -> ()
          }
          frame #7 {
            n792 = Get Date/Time In Seconds() -> (seconds since 1Jan1904=w833:timestamp)
            n793 = Format Into String(format string="%<%I:%M:%S:%p %d:%B:%Y>T", w833) -> (resulting string=w832:string)  [unwired: 2 in, 1 out]
            n794 = local write "TEMPERATURE CALIBRATION"(w832) -> ()
          }
          frame #8 {
            n795 = local write "Save Button"(TRUE ("Save Button")) -> ()
          }
        }
      }
      event "Temperature Continue Step 6": Value Change {
        n796 = event-data() -> ()  [unwired: 1 in, 6 out]
        n797 = stacked-sequence {
          frame #0 {
            n798 = stacked-sequence {
              frame #0 {
                n799 = Wait (ms)(milliseconds to wait=u32 1000) -> ()  [unwired: 1 out]
              }
              frame #1 {
              }
              frame #2 {
              }
              frame #3 {
                # "CAL;A1;<true_T>"
                n800 = local write "Due Write"("CAL;A1;60" ("Command")) -> ()
              }
              frame #4 {
                n801 = Wait (ms)(milliseconds to wait=u32 1000) -> ()  [unwired: 1 out]
              }
              frame #5 {
                # "CAL;A1;<true_T>"
                n802 = local write "Due Write"("CAL;A1;60" ("Command")) -> ()
              }
            }
          }
          frame #1 {
            n803 = local read "Sensor value"() -> (→"Air 60deg temp":dbl)
          }
          frame #2 {
          }
          frame #3 {
          }
          frame #4 {
          }
          frame #5 {
          }
          frame #6 {
            # "CAL;END"
          }
          frame #7 {
            n804 = local read "Temperature diff"() -> (w842:dbl)
            n805 = local read "Air 60deg temp"() -> (w841:dbl)
            n806 = local read "Air 0deg temp"() -> (w840:dbl)
            n807 = Add(x=w841, y=w842) -> (x+y=w849:dbl)
            n808 = Subtract(x=w841, y=w842) -> (x-y=w848:dbl)
            n809 = Add(x=w840, y=w842) -> (x+y=w847:dbl)
            n810 = Subtract(x=w840, y=w842) -> (x-y=w846:dbl)
            n811 = In Range and Coerce(upper limit=w849, x=w841, lower limit=w848) -> (In Range?=w845:bool)  [unwired: 1 out]
            n812 = In Range and Coerce(upper limit=w847, x=w840, lower limit=w846) -> (In Range?=w844:bool)  [unwired: 1 out]
            n813 = And(x=w845, y=w844) -> (x .and. y?=w843:bool)
            n814 = case shown="True" w843 {
              frame False {
                n815 = property on="Accept & Save Air Temperature step 4" class="Bool (strict)"("DisabledEnum"=T19."Disabled" ("Disabled")) -> ()  [unwired: 2 in, 2 out]